vi "Transconductance state machine.vi"() -> ()   [LabVIEW 2016]
uses:
  <vilib>/Analysis/3filter.llb/Filter Passband Type.ctl
  <vilib>/Analysis/6fits.llb/Remove Outliers (Range).vi
  <vilib>/Analysis/3filter.llb/Chebyshev Filter (DBL).vi
  <vilib>/Analysis/NI_AALPro.lvlib
  <vilib>/Analysis/NI_AALBase.lvlib
  <vilib>/Analysis/NI_AAL_SigProc.lvlib
panel:
  in  "Tab Control 2":T1(tab)
  out "Conductance curve\nvertical line cut":cluster{dbl[], "Decimated Array":dbl[]}(graph)
  out "B field (T)":dbl
  out "Transcond curve\nhorizontal line cut":cluster{dbl[], dbl[]}(graph)
  out "Vsg (V)":dbl format="%#_6p"
  in  "Load data":bool
  in  "Refresh":bool
  in  "Tab Control":T2(tab)=enum."Flatten Transconductance"
  in  "index":T3={"N1 (x axis)"=3, "N2"=19, "N3"=4, "N4"=5, "V1"=8, "V2"=4, "V3"=10, "V4"=13, "CURRENT"=6, "Vsg"=1}
  in  "File or Folder Path":path=path "G:/My Drive/ansom/Data/MNK/SA03018F.20180426/3 - sweep B, Vsg lockin, superlattice"
  out "original cond":T4(graph)
  out "Comments":string="IGOR\nX// Date: 5/2/2018 10:25 PM\nX// B=0T to 18T, 0.03 T/min\nX// T=40mK\nX// sweep Vsg -10mV --> 60mV, 50uV step\nX// Vsg=1.1V\nX// \nX// lockin settings:\nX// time constant =100ms\nX// order=2\nX// Fs=13000\nX// #s=1000\nX// \nX// both\nX// \nX// lockin:\nX// 0: 4, voltage V+\nX// 1: 5,  current 50uV AC 270uV DC, 13 Hz\nX// 2: 7,voltage V-\nX// 3: 3, current, drain\nX// 4: 2,\nX// 5: 1, \nX// `INDEX`<WavesIndex_In_2>\n\nX//   <Side_Gate>1</Side_Gate>\n\nX//   <Current>6</Current>\n\nX//   <Voltage_1>8</Voltage_1>\n\nX//   <Voltage_2>4</Voltage_2>\n\nX//   <B_Field>3</B_Field>\n\nX//   <Voltage>true</Voltage>\n\nX// </WavesIndex_In_2>`INDEX`\n\n\n\n\n\n\n\n\n\n\n\n\n\n\n\n\n\n\n\n\n\n\n\n\n\n\n\n\n\n\n\n\n\n\n\n\n\n\n\n\n\n\n\n\n\n\n\n\n\n\n\n\n\n\n\n\n\n\nX \nX Display/R 'time.SA03018F.20180502.000001'\nX AppendToGraph 'Vsg.SA03018F.20180502.000001'\nX AppendToGraph 'T.SA03018F.20180502.000001'\nX AppendToGraph 'B.SA03018F.20180502.000001'\nX AppendToGraph 'X0.SA03018F.20180502.000001'\nX AppendToGraph 'Y0.SA03018F.20180502.000001'\nX AppendToGraph 'X1.SA03018F.20180502.000001'\nX AppendToGraph 'Y1.SA03018F.20180502.000001'\nX AppendToGraph 'X2.SA03018F.20180502.000001'\nX AppendToGraph 'Y2.SA03018F.20180502.000001'\nX AppendToGraph 'X3.SA03018F.20180502.000001'\nX AppendToGraph 'Y3.SA03018F.20180502.000001'\nX AppendToGraph 'X4.SA03018F.20180502.000001'\nX AppendToGraph 'Y4.SA03018F.20180502.000001'\nX AppendToGraph 'X5.SA03018F.20180502.000001'\nX AppendToGraph 'Y5.SA03018F.20180502.000001'\nX AppendToGraph 'B_rate.SA03018F.20180502.000001'\nX AppendToGraph 'R4t(e2/h).SA03018F.20180502.000001'\nX AppendToGraph 'axis1.SA03018F.20180502.000001'\nX AppendToGraph 'axis2.SA03018F.20180502.000001'\nX AppendToGraph '20.SA03018F.20180502.000001'\nX AppendToGraph '21.SA03018F.20180502.000001'\nX AppendToGraph '22.SA03018F.20180502.000001'\nX AppendToGraph '23.SA03018F.20180502.000001'\nX AppendToGraph '24.SA03018F.20180502.000001'\nX AppendToGraph '25.SA03018F.20180502.000001'\nX AppendToGraph '26.SA03018F.20180502.000001'\nX AppendToGraph '27.SA03018F.20180502.000001'\nX Label bottom \"x label\"\nX Label left \"y label\"\nX ModifyGraph rgb('time.SA03018F.20180502.000001')=(65280,0,0)\nX ModifyGraph rgb('Vsg.SA03018F.20180502.000001')=(65280,12288,0)\nX ModifyGraph rgb('T.SA03018F.20180502.000001')=(65280,24576,0)\nX ModifyGraph rgb('B.SA03018F.20180502.000001')=(65280,38400,0)\nX ModifyGraph rgb('X0.SA03018F.20180502.000001')=(65280,50688,0)\nX ModifyGraph rgb('Y0.SA03018F.20180502.000001')=(65280,62976,0)\nX ModifyGraph rgb('X1.SA03018F.20180502.000001')=(55808,65280,0)\nX ModifyGraph rgb('Y1.SA03018F.20180502.000001')=(43520,65280,0)\nX ModifyGraph rgb('X2.SA03018F.20180502.000001')=(29696,65280,0)\nX ModifyGraph rgb('Y2.SA03018F.20180502.000001')=(17408,65280,0)\nX ModifyGraph rgb('X3.SA03018F.20180502.000001')=(5120,65280,0)\nX ModifyGraph rgb('Y3.SA03018F.20180502.000001')=(0,65280,7168)\nX ModifyGraph rgb('X4.SA03018F.20180502.000001')=(0,65280,20992)\nX ModifyGraph rgb('Y4.SA03018F.20180502.000001')=(0,65280,33280)\nX ModifyGraph rgb('X5.SA03018F.20180502.000001')=(0,65280,45568)\nX ModifyGraph rgb('Y5.SA03018F.20180502.000001')=(0,65280,57856)\nX ModifyGraph rgb('B_rate.SA03018F.20180502.000001')=(0,60928,65280)\nX ModifyGraph rgb('R4t(e2/h).SA03018F.20180502.000001')=(0,47104,65280)\nX ModifyGraph rgb('axis1.SA03018F.20180502.000001')=(0,34816,65280)\nX ModifyGraph rgb('axis2.SA03018F.20180502.000001')=(0,22528,65280)\nX ModifyGraph rgb('20.SA03018F.20180502.000001')=(0,10240,65280)\nX ModifyGraph rgb('21.SA03018F.20180502.000001')=(2048,0,65280)\nX ModifyGraph rgb('22.SA03018F.20180502.000001')=(15872,0,65280)\nX ModifyGraph rgb('23.SA03018F.20180502.000001')=(28160,0,65280)\nX ModifyGraph rgb('24.SA03018F.20180502.000001')=(40448,0,65280)\nX ModifyGraph rgb('25.SA03018F.20180502.000001')=(52736,0,65280)\nX ModifyGraph rgb('26.SA03018F.20180502.000001')=(65280,0,64512)\nX ModifyGraph rgb('27.SA03018F.20180502.000001')=(65280,0,52224)\nX Legend/C/N=text0/J \"\\\\s('time.SA03018F.20180502.000001') time\\r\\\\s('Vsg.SA03018F.20180502.000001') Vsg\\r\\\\s('T.SA03018F.20180502.000001') T\\r\\\\s('B.SA03018F.20180502.000001') B\\r\\\\s('X0.SA03018F.20180502.000001') X0\\r\\\\s('Y0.SA03018F.20180502.000001') Y0\\r\\\\s('X1.SA03018F.20180502.000001') X1\\r\\\\s('Y1.SA03018F.20180502.000001') Y1\\r\\\\s('X2.SA03018F.20180502.000001') X2\\r\\\\s('Y2.SA03018F.20180502.000001') Y2\\r\\\\s('X3.SA03018F.20180502.000001') X3\\r\\\\s('Y3.SA03018F.20180502.000001') Y3\\r\\\\s('X4.SA03018F.20180502.000001') X4\\r\\\\s('Y4.SA03018F.20180502.000001') Y4\\r\\\\s('X5.SA03018F.20180502.000001') X5\\r\\\\s('Y5.SA03018F.20180502.000001') Y5\\r\\\\s('B_rate.SA03018F.20180502.000001') B_rate\\r\\\\s('R4t(e2/h).SA03018F.20180502.000001') R4t (e2/h)\\r\\\\s('axis1.SA03018F.20180502.000001') axis 1\\r\\\\s('axis2.SA03018F.20180502.000001') axis 2\"\nX ModifyGraph mirror(bottom)=1\nX ModifyGraph width=216\nX ModifyGraph height={Aspect,0.6}\nX ModifyGraph Log(bottom)=0\nX ModifyGraph Log(left)=0\nX \n"
  in  "offset":i32
  in  "length":i32=1000
  in  "conductance range":dbl[](array[numeric])=[-1.0, 20.0]
  in  "Filter?":bool=TRUE
  in  "low cutoff freq: fh 2":dbl=0.05 format="%0.2f"
  in  "restrict range?":bool=TRUE
  in  "dy/dx vs x":bool=TRUE
  in  "derivative points":dbl=20.0
  out "Cond intensity":dbl[][](graph)
  out "Conductance":T4(graph)
  in  "offset cond (horizontal)":dbl=0.001
  out "Transconductance":T4(graph)
  out "Transcond Intensity":dbl[][](graph)
  in  "offset trans (vertical)":dbl
  out "modified transconductance":T4(graph)
  in  "threshold":dbl=25.0 format="%0.2f"
  in  "width":i32=20 min=3
  in  "X Low":dbl=-0.1 format="%#_6p"
  in  "X High":dbl=0.1 format="%#_6p"
  out "Flattened Transconductance":dbl[][](graph)
  in  "manual offset array":dbl[](array[numeric])
  out "number of curves":i32
  in  "Stop":bool
  # "Conductance curve, select using cursor on transconductance \nintensity plot"
  # "choose N1 to be the B field, or other slow parameter\nfor intensity plots"
  # "creates conductnace plot\ny axis: current/(V1-V2)\nx axis: Vsg"
  # "To apply changes press the 'Refresh' button"
  # "Modify conductance data"
  # "Transconductnace derivative parameters"
  # "Peak finding parameters for \nflattening transconductance"
  # "Interpolating parameters"
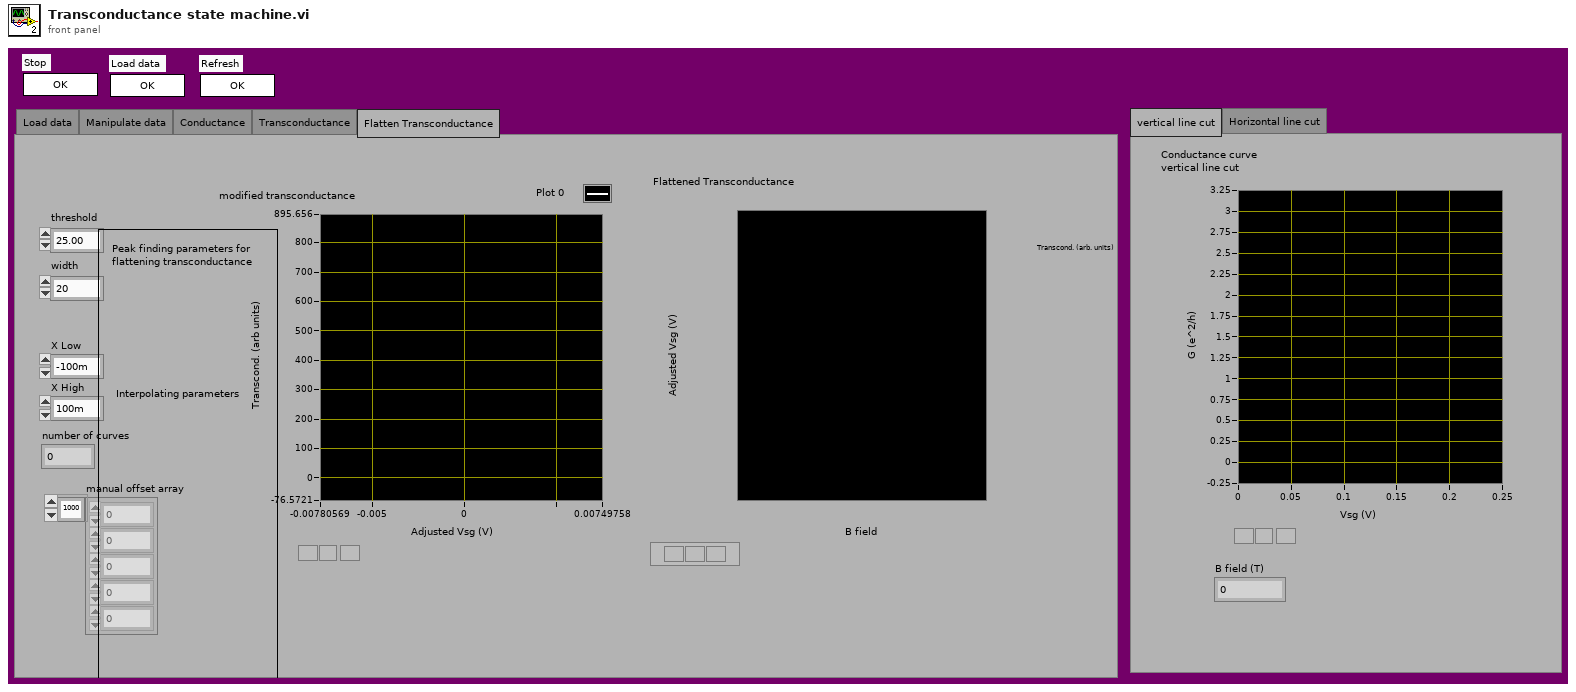
[diagram p1: front panel]
types:
  T1 = enum32{"vertical line cut", "Horizontal line cut"}
  T2 = enum32{"Load data", "Manipulate data", "Conductance", "Transconductance", "Flatten Transconductance"}
  T3 = cluster{"N1 (x axis)":i32, "N2":i32, "N3":i32, "N4":i32, "V1":i32, "V2":i32, "V3":i32, "V4":i32, "CURRENT":i32, "Vsg":i32}
  T4 = cluster{"Vfast":dbl[], "Decimated Array":dbl[]}[]
  T5 = enum32{"invalid app kind", "Development System", "Run Time System", "Student Edition", "Embedded LabVIEW", "Evaluation", "Custom"}
  T6 = enum32{"Invalid", "Standard", "Closed", "Hidden", "Minimized", "Maximized"}
  T7 = typedef "NI_AALBase.lvlib/Filter Passband Type.ctl" = enum32{"Lowpass", "Highpass", "Bandpass", "Bandstop"}
  T8 = cluster{"Core":cluster{"Current VI Reference":refnum<vi>, "Close Panel on Exit?":bool}, "Original Conductance":cluster{"Vfast":dbl[], "Decimated Array":dbl[]}[], "Modified Conductance":cluster{"Vfast":dbl[], "Decimated Array":dbl[]}[], "Transconductance":cluster{"Vfast":dbl[], "Decimated Array":dbl[]}[], "Modified Transconductance":cluster{"Vfast":dbl[], "Decimated Array":dbl[]}[], "Cond Intensity":dbl[][], "Transcond Intensity":dbl[][], "N Array":cluster{"N1":dbl, "N2":dbl, "N3":dbl, "N4":dbl}[], "N1 (B field)":dbl[], "Vsg offset and mult":cluster{dbl, dbl}, "B offset and mult":cluster{dbl, dbl}, "number of curves":i32, "cursor plot":i32, "curson index":i32}
  T9 = cluster{"N1":dbl, "N2":dbl, "N3":dbl, "N4":dbl}[]
  T10 = cluster{"Current VI Reference":refnum<vi>, "Close Panel on Exit?":bool}
  T11 = typedef "LVOffsetAndMultiplierTypeDef.ctl" = cluster{"Offset":dbl, "Multiplier":dbl}
  T12 = cluster{"Decimated Array":dbl[], "Decimated Array":dbl[]}
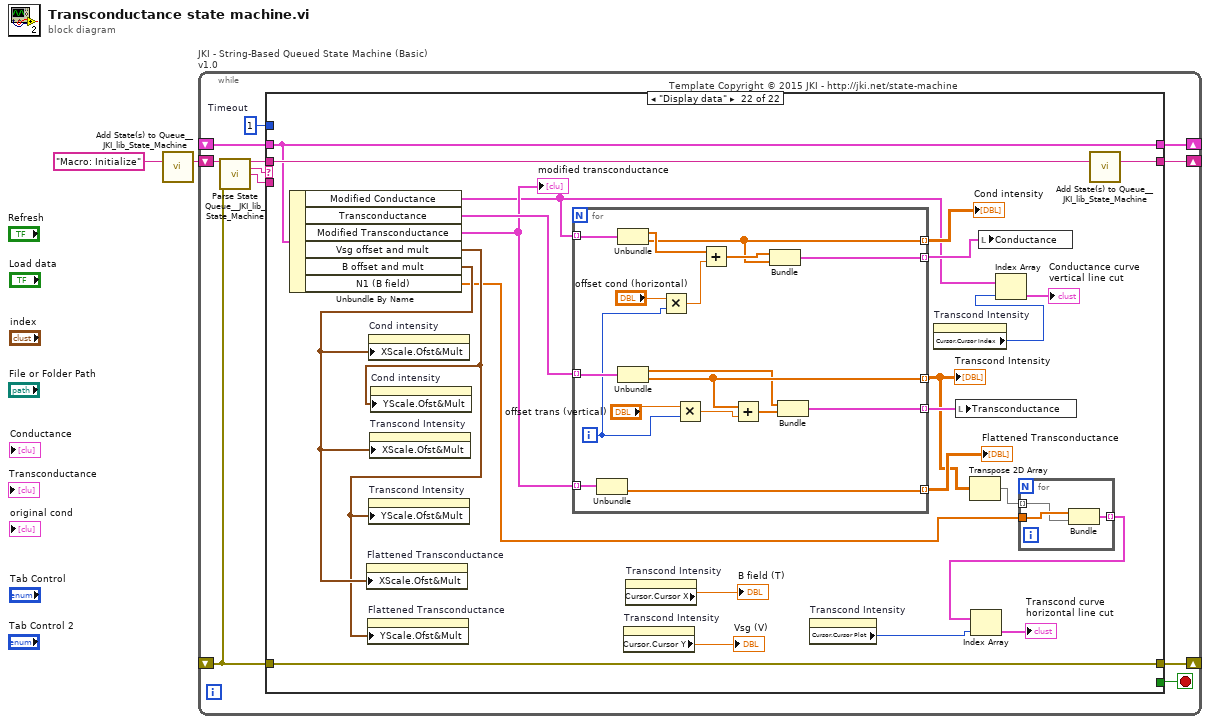
[diagram p0: block diagram]
diagram:
  n1 = call <vilib>:"Add State(s) to Queue__JKI_lib_State_Machine.vi"("State(s) in (\"\")"="Macro: Initialize") -> ("States Out"=w2:string)  [unwired: 14 in]
  n2 = while "JKI - String-Based Queued State Machine (Basic) v1.0" {
    shift-right: [w6] -> _
    shift-left: _ -> [w5]
    shift-right: [w9] -> _
    shift-left: _ -> [w3]
    shift-right: [w8] -> _
    shift-left: w2 -> [w10]
    stop <- w7 stop-if-true
    w4 = 1  # Timeout
    # "Template Copyright © 2015 JKI - http://jki.net/state-machine"
    n3 = call <vilib>:"Parse State Queue__JKI_lib_State_Machine.vi"("State Queue"=w10, "Error In (no error)"=w3) -> ("Remaining States"=w12:string, "Current State"=w13:string, "Arguments"=w11:string)  [unwired: 11 in]
    n4 = case shown="\"Display data\"" w13 {
      selector: w13 -> [_ _ w82 _ _ _ _ _ _ _ _ _ _ _ _ _ _ _ _ _ _ _]
      tunnel: w12 -> [w20 w81 w86 w104 w110 w115 w119 w137 w143 w147 w155 w161 w172 w198 w203 w213 w217 w256 w269 w298 w316 w357]
      tunnel: w11 -> [_ _ _ _ _ _ _ _ _ _ _ w156 w166 _ _ _ _ _ _ _ _ _]
      tunnel: w5 -> [w18 w78 w84 w95 w107 w113 w116 _ w138 w144 w152 w159 w168 w195 w200 w210 w214 w223 w261 w294 w313 w354]
      tunnel: [w17 w79 w88 w101 errorcluster {"status"=FALSE, "code"=0, "source"=""} ("error out") w112 w117 w134 w139 w145 w153 w157 w169 w196 w201 w211 w215 w254 w267 w296 w314 w355] -> w9
      tunnel: w3 -> [w16 w79 w87 w101 w106 w112 w117 w134 w140 w145 w153 w158 w170 w196 w201 w211 w215 w254 w267 w296 w314 w355]
      tunnel: [w19 w80 w85 w103 w109 w114 w118 w136 w142 w146 w154 w160 w171 w197 w202 w212 w216 w255 w268 w297 w315 w356] -> w8
      tunnel: [_ _ _ _ _ TRUE _ _ _ _ _ _ _ _ _ _ _ _ _ _ _ _] -> w7
      tunnel: [w15 w78 w84 w102 w107 w113 w116 w135 w138 w144 w150 w159 w168 w195 w200 w210 w214 w251 w259 w292 w312 w354] -> w6
      tunnel: w4 -> [w14 _ _ _ _ _ _ _ _ _ _ _ _ _ _ _ _ _ _ _ _ _]
      frame "", "Event Structure", "Idle" {
        # "executes when the state queue is empty"
        n5 = event shown="[3] \"Refresh\": Value Change" {
          selector: _ -> [_ _ _ _ _ _ _ _]
          dyn-events: _ -> [_ _ _ _ _ _ _ _]
          timeout: w14 -> [_ _ _ _ _ _ _ _]
          tunnel: w20 -> [w30 w35 w40 w45 w46 w56 w69 w77]
          tunnel: [w29 w34 w39 w44 w47 w55 w68 w76] -> w19
          tunnel: w18 -> [w26 w32 w37 w42 w49 w57 w67 w74]
          tunnel: [w28 w33 w38 w43 w48 w54 w62 w75] -> w17
          tunnel: w16 -> [w28 w33 w38 w43 w48 w54 w62 w75]
          tunnel: [w25 w32 w37 w42 w49 w57 w67 w74] -> w15
          event Timeout {
            n6 = event-data() -> ()  [unwired: 1 in, 1 out]
            n7 = local read "original cond"() -> (w22:T4)
            n8 = property on="Transcond Intensity" class="IntGraph (strict)"() -> ("Cursor.Cursor Index"=w23:i32)  [unwired: 2 in, 2 out]
            n9 = property on="Transcond Intensity" class="IntGraph (strict)"() -> ("Cursor.Cursor Plot"=w24:i32)  [unwired: 2 in, 2 out]
            n10 = Array Size(array=w22) -> (size(s)=w21:i32)
            n11 = Bundle By Name(cluster=w26, "cursor plot"=w24, "curson index"=w23, "number of curves"=w21) -> (w25:T8)
            n12 = call <vilib>:"Add State(s) to Queue__JKI_lib_State_Machine.vi"("State(s) in (\"\")"=w30, "State(s) at Back (\"\")"="Display data" ("State(s) at Back (\"\")")) -> ("States Out"=w29:string)  [unwired: 13 in]
          }
          event "Stop": Value Change {
            # "Exit Button Value Change (pressed) Event\n(this executes Macro: Exit to terminate the VI)"
            n13 = event-data() -> ()  [unwired: 1 in, 1 out]
            n14 = call <vilib>:"Add State(s) to Queue__JKI_lib_State_Machine.vi"("State(s) in Front (\"\")"="Macro: Exit", "State(s) in (\"\")"=w35) -> ("States Out"=w34:string)  [unwired: 13 in]
          }
          event "Load data": Value Change {
            # "Load data using 'Calculate conductance ITX.vi'\n\nmust set the folder path and the index"
            n15 = event-data() -> ()  [unwired: 1 in, 1 out]
            n16 = call <vilib>:"Add State(s) to Queue__JKI_lib_State_Machine.vi"("State(s) in Front (\"\")"="Load data", "State(s) in (\"\")"=w40) -> ("States Out"=w39:string)  [unwired: 13 in]
          }
          event "Refresh": Value Change {
            # "Refresh graphs with any changes in manipulate data tab\n\nwill also display the data in the 'original cond' graph if no\nnew data has been loaded since starting the program"
            n17 = event-data() -> ()  [unwired: 1 in, 1 out]
            n18 = call <vilib>:"Add State(s) to Queue__JKI_lib_State_Machine.vi"("State(s) in Front (\"\")"="Manipulate data", "State(s) in (\"\")"=w45) -> ("States Out"=w44:string)  [unwired: 13 in]
          }
          event "Flattened Transconductance": Cursor Move {
            n19 = event-data() -> ()  [unwired: 1 in, 9 out]
            n20 = property on="Flattened Transconductance" class="IntGraph (strict)"() -> ("Cursor.Cursor Index"=w51:i32, "Cursor.Cursor Plot"=w50:i32)  [unwired: 2 in, 2 out]
            n21 = property on="Transcond Intensity" class="IntGraph (strict)"("Cursor.Cursor Index"=w51, "Cursor.Cursor Plot"=w50) -> ()  [unwired: 2 in, 2 out]
            n22 = call <vilib>:"Add State(s) to Queue__JKI_lib_State_Machine.vi"("State(s) in (\"\")"=w46) -> ("States Out"=w47:string)  [unwired: 14 in]
          }
          event "Cond intensity": Cursor Move {
            n23 = event-data() -> ()  [unwired: 1 in, 9 out]
            n24 = property on="Cond intensity" class="IntGraph (strict)"() -> ("Cursor.Cursor Index"=w53:i32, "Cursor.Cursor Plot"=w52:i32)  [unwired: 2 in, 2 out]
            n25 = property on="Transcond Intensity" class="IntGraph (strict)"("Cursor.Cursor Index"=w53, "Cursor.Cursor Plot"=w52) -> ()  [unwired: 2 in, 2 out]
            n26 = call <vilib>:"Add State(s) to Queue__JKI_lib_State_Machine.vi"("State(s) in (\"\")"=w56) -> ("States Out"=w55:string)  [unwired: 14 in]
          }
          event "Transcond Intensity": Cursor Move {
            # "Change visible tab in line cut tab control when the cursor on the transconductance intensity plot is moved\nmoving the vertical cursor shows the vertical line cut, moving the horizontal cursor shows the horizontal line cut"
            n27 = event-data() -> ("CursIdx"=w63:i32, "PlotIdx"=w64:i32)  [unwired: 1 in, 7 out]
            n28 = Unbundle By Name(w67) -> ("curson index"=w66:i32, "cursor plot"=w65:i32)
            n29 = Not Equal?(x=w66, y=w63) -> (x != y?=w61:bool)
            n30 = Not Equal?(x=w65, y=w64) -> (x != y?=w60:bool)
            n31 = And(x=w61, y=w60) -> (x .and. y?=w59:bool)
            n32 = case shown="True" w59 {
              tunnel: [T1."vertical line cut" ("Tab Control 2") T1."Horizontal line cut" ("Tab Control 2")] -> w58
              frame False {
              }
              frame True {
              }
            }
            n33 = local write "Tab Control 2"(w58) -> ()
            n34 = call <vilib>:"Add State(s) to Queue__JKI_lib_State_Machine.vi"("State(s) in (\"\")"=w69) -> ("States Out"=w68:string)  [unwired: 14 in]
          }
          event Panel Close? {
            # "Discard the event because we'll close the front panel ourselves in Macro: Exit"
            # "Close Panel button (pressed) Event\n(this executes Macro: Exit to terminate the VI)"
            n35 = event-data() -> ()  [unwired: 1 in, 1 out]
            n36 = call <vilib>:"Add State(s) to Queue__JKI_lib_State_Machine.vi"("State(s) in Front (\"\")"="Macro: Exit", "State(s) in (\"\")"=w77) -> ("States Out"=w76:string)  [unwired: 13 in]
            n37 = event-data("Discard?"=TRUE) -> ()  [unwired: 1 in, 1 out]
          }
        }
      }
      frame "---------- Core ----------" {
        # "Do not put any code in this frame.\n(it is a separator no-op)"
        n38 = call <vilib>:"Add State(s) to Queue__JKI_lib_State_Machine.vi"("State(s) in (\"\")"=w81) -> ("States Out"=w80:string)  [unwired: 14 in]
      }
      frame Default {
        w91 = 42 items=["No error", "Argument error", "Memory is full", "Out of zone", "End of file", "File already open", "Generic file I/O error", "File not found", "File permission error", "Disk is full", "Duplicate path", "Too many files open", "System feature not enabled", "Resource file not found", "Cannot add resource", "Resource not found", "Image not found", "Image memory error", "Pen does not exist", "Config type invalid", "Config token not found", "Config parse error", "Config memory error", "Bad external code format", "Bad external code offset", "External code not present", "Null window", "Destroy window error", "Null menu", "Print aborted", "Bad print record", "Print driver error", "Windows error during printing", "Memory error during printing", "Print dialog error", "Generic print error", "Invalid device refnum", "Device not found", "Device parameter error", "Device unit error", "Cannot open device", "Device call aborted", "Generic error", "Cancelled by user", "Object ID too low", "Object ID too high", "Object not in heap", "Unknown heap", "Unknown object (invalid DefProc)", "Unknown object (DefProc not in table)", "Message out of range", "Invalid (null) method", "Unknown message", "Manager call not supported", "Bad address", "Network operation in progress", "Network operation timed out", "Connection is busy", "Network attribute not supported", "Network error", "Address in use", "System out of memory", "Connection aborted", "Connection refused", "Not connected", "Already connected", "Connection closed", "Initialization error (interapplication manager)", "Bad occurrence", "Wait on unbound occurrence handler", "Occurrence queue overflow", "Datalog type conflict", "Unused", "Unrecognized type (interapplication manager)", "Memory corrupt", "Failed to make temporary DLL", "Old CIN version", "Drag socket not found", "Failed to load drop-object", "Failed to register OLE object", "Failed to release OLE object", "Format specifier type mismatch", "Unknown format specifier", "Too few format specifiers", "Too many format specifiers", "Scan failed", "Newer CIN version", "Error converting to variant", "Runtime menu error", "Password tampered", "Variant attribute not found", "Incompatible variant data type", "Event data is not available", "Event Store is not present", "Occurrence is not found", "Event Queue is not created", "Event info is not available", "Refnum passed is NULL", "Error retrieving Class GUID", "Error retrieving CoClass GUID", "Error retrieving TypeLib GUID.", "Bad built application magic bytes.", "Specific driver is different from the specific driver associated with the Logical Name.", "There is no session opened to the class driver.", "Max Error", "MAX - Error with config objects", "MAX - Error loading configuration", "MAX - Group not supported"]
        # "Current State"
        # "Do not delete, rename, or modify this frame.\n(this is used to capture unhandled states and typos)"
        # "Handle mistyped state name (developer tool)"
        n39 = Format Into String(format string="Software Exception: Unhandled State \"%s\"." ("message"), error in=w87, w82) -> (resulting string=w90:string, error out=w89:errorcluster)  [unwired: 1 in]
        n40 = call <vilib>:"Error Cluster From Error Code.vi"("show call chain? (False)"=TRUE, "error in (no error)"=w89, "error message (\"\")"=w90, "error code (0)"=w91) -> ("error out"=w88:errorcluster)  [unwired: 5 in]
        n41 = call <vilib>:"Add State(s) to Queue__JKI_lib_State_Machine.vi"("State(s) in (\"\")"=w86) -> ("States Out"=w85:string)  [unwired: 14 in]
      }
      frame "Initialize Core Data" {
        # "Do not delete, rename, or modify this frame.\n(this is used to determine panel behavior on exit)"
        # "originally closed?"
        # "exe?"
        # "If panel starts closed or is an EXE, then close it when we exit"
        n42 = property class="VI"() -> ("Front Panel.Open"=w100:bool)  [unwired: 2 in, 2 out]
        n43 = property class="App"() -> ("App.Kind"=w99:T5)  [unwired: 2 in, 2 out]
        n44 = control-ref of="Current VI Reference"() -> (w93:refnum<vi>)
        n45 = Not(x=w100) -> (.not. x?=w97:bool)
        n46 = Equal?(x=w99, y=T5."Run Time System" ("Application:Kind")) -> (x = y?=w96:bool)
        n47 = Or(x=w97, y=w96) -> (x .or. y?=w94:bool)
        n48 = Bundle By Name(cluster=w95, "Core.Current VI Reference"=w93, "Core.Close Panel on Exit?"=w94) -> (w102:T8)
        n49 = call <vilib>:"Add State(s) to Queue__JKI_lib_State_Machine.vi"("State(s) in (\"\")"=w104) -> ("States Out"=w103:string)  [unwired: 14 in]
      }
      frame "Error Handler" {
        # "Unhandled Error -- Display it"
        # "Handle any errors here.\nYou can also output any states to clean-up after errors occur"
        # "Clear error"
        n50 = call <vilib>:"General Error Handler.vi"("error in (no error)"=w106) -> ()  [unwired: 10 in, 5 out]
        n51 = call <vilib>:"Add State(s) to Queue__JKI_lib_State_Machine.vi"("State(s) in Front (\"\")"="/* Post Error States", "State(s) in (\"\")"=w110) -> ("States Out"=w109:string)  [unwired: 13 in]
      }
      frame "Exit" {
        # "Do not put any code in this frame.\n(No errors that occur here will be handled.)"
        n52 = call <vilib>:"Add State(s) to Queue__JKI_lib_State_Machine.vi"("State(s) in (\"\")"=w115) -> ("States Out"=w114:string)  [unwired: 14 in]
      }
      frame "---------- Data ----------" {
        # "Do not put any code in this frame.\n(It is a separator no-op. You can make a copy of this frame to create a new Data frame)"
        n53 = call <vilib>:"Add State(s) to Queue__JKI_lib_State_Machine.vi"("State(s) in (\"\")"=w119) -> ("States Out"=w118:string)  [unwired: 14 in]
      }
      frame "Data: Initialize" {
        w120 = 0  # curson index
        w121 = 0  # cursor plot
        w122 = T4 []  # Modified Transconductance
        w123 = 0  # number of curves
        w124 = cluster{dbl, dbl} {0.0, 0.0}  # B offset and mult
        w125 = cluster{dbl, dbl} {0.0, 0.0}  # Vsg offset and mult
        w126 = dbl[] []  # N1 (B field)
        w127 = T4 []  # Modified Conductance
        w128 = T9 [{"N1"=0.1054, "N2"=0.0, "N3"=7.167371706088133e-06, "N4"=1.53337376832391e-06}, {"N1"=0.2744, "N2"=0.0, "N3"=7.516017465840743e-06, "N4"=1.870780961155766e-06}, {"N1"=0.4429, "N2"=0.0, "N3"=7.164956665698316e-06, "N4"=2.24365763977575e-06}, {"N1"=0.6118, "N2"=0.0, "N3"=7.47503008732585e-06, "N4"=2.509786953376164e-06}, {"N1"=0.78, "N2"=0.0, "N3"=7.582119269367365e-06, "N4"=1.865776048611999e-06}, {"N1"=0.9496, "N2"=0.0, "N3"=7.367991857506643e-06, "N4"=2.698521756661702e-06}, {"N1"=1.1176, "N2"=0.0, "N3"=7.227789507339006e-06, "N4"=2.57461130832219e-06}, {"N1"=1.2843, "N2"=0.0, "N3"=7.066841533109455e-06, "N4"=3.048492296414582e-06}, {"N1"=1.4544, "N2"=0.0, "N3"=6.956050970108828e-06, "N4"=3.922270862071821e-06}, {"N1"=1.6231, "N2"=0.0, "N3"=7.236120895401367e-06, "N4"=3.382292471609201e-06}, {"N1"=1.7923, "N2"=0.0, "N3"=7.409928531135188e-06, "N4"=2.980502224034656e-06}, {"N1"=1.9608, "N2"=0.0, "N3"=7.465240274926555e-06, "N4"=2.567980193012299e-06}, {"N1"=2.1296, "N2"=0.0, "N3"=7.67996705698243e-06, "N4"=2.820594776222847e-06}, {"N1"=2.2974, "N2"=0.0, "N3"=7.462806473700619e-06, "N4"=3.043330294253364e-06}, {"N1"=2.4668, "N2"=0.0, "N3"=7.436808347763807e-06, "N4"=2.755707470732885e-06}, {"N1"=2.6348, "N2"=0.0, "N3"=6.62119487806683e-06, "N4"=3.938204565752024e-06}, {"N1"=2.8044, "N2"=0.0, "N3"=7.474110207381518e-06, "N4"=2.685132266272008e-06}, {"N1"=2.9727, "N2"=0.0, "N3"=7.467721317681889e-06, "N4"=2.490711666292731e-06}, {"N1"=3.1413, "N2"=0.0, "N3"=7.373756967263423e-06, "N4"=3.233877080828954e-06}, {"N1"=3.3108, "N2"=0.0, "N3"=7.665479000670658e-06, "N4"=2.656474229977507e-06}, {"N1"=3.4787, "N2"=0.0, "N3"=7.590986063837561e-06, "N4"=2.372468698283599e-06}, {"N1"=3.6474, "N2"=0.0, "N3"=7.403426727936138e-06, "N4"=2.492719733694041e-06}, {"N1"=3.8169, "N2"=0.0, "N3"=7.673375229594714e-06, "N4"=2.203309425429715e-06}, {"N1"=3.9853, "N2"=0.0, "N3"=7.235339121315365e-06, "N4"=2.455197981754483e-06}, {"N1"=4.1517, "N2"=0.0, "N3"=7.588783683002382e-06, "N4"=2.171945449692774e-06}, {"N1"=4.3221, "N2"=0.0, "N3"=7.448410925151985e-06, "N4"=2.89278994654584e-06}, {"N1"=4.4909, "N2"=0.0, "N3"=7.559811002403063e-06, "N4"=2.32906566750442e-06}, {"N1"=4.6597, "N2"=0.0, "N3"=7.589944875648538e-06, "N4"=2.522315779577562e-06}, {"N1"=4.828, "N2"=0.0, "N3"=7.486560787096485e-06, "N4"=2.673968837700548e-06}, {"N1"=4.9975, "N2"=0.0, "N3"=7.764068992589737e-06, "N4"=2.470810112270278e-06}, {"N1"=5.1656, "N2"=0.0, "N3"=7.515430091426793e-06, "N4"=2.347750168384078e-06}, {"N1"=5.3343, "N2"=0.0, "N3"=7.61778177581086e-06, "N4"=2.441280739349988e-06}, {"N1"=5.5028, "N2"=0.0, "N3"=7.648092365254961e-06, "N4"=2.50884391552613e-06}, {"N1"=5.6718, "N2"=0.0, "N3"=7.607187802074639e-06, "N4"=2.479224506195392e-06}, {"N1"=5.8408, "N2"=0.0, "N3"=7.675790190344634e-06, "N4"=2.243726367409315e-06}, {"N1"=6.0093, "N2"=0.0, "N3"=7.5989905280867e-06, "N4"=2.339493694595715e-06}, {"N1"=6.1776, "N2"=0.0, "N3"=7.946377320613181e-06, "N4"=2.179171604450671e-06}, {"N1"=6.3464, "N2"=0.0, "N3"=7.788145582711778e-06, "N4"=1.980962373666305e-06}, {"N1"=6.5143, "N2"=0.0, "N3"=7.613597487476077e-06, "N4"=2.305590643717492e-06}, {"N1"=6.6841, "N2"=0.0, "N3"=7.704173394418159e-06, "N4"=2.229928539054291e-06}, {"N1"=6.8524, "N2"=0.0, "N3"=7.719187746028896e-06, "N4"=1.959910122360407e-06}, {"N1"=7.0199, "N2"=0.0, "N3"=7.54069778807839e-06, "N4"=2.119395007811887e-06}, {"N1"=7.1892, "N2"=0.0, "N3"=7.780578976603794e-06, "N4"=2.065252716472169e-06}, {"N1"=7.359, "N2"=0.0, "N3"=7.850755995736213e-06, "N4"=2.026777225217505e-06}, {"N1"=7.5271, "N2"=0.0, "N3"=7.948557406193015e-06, "N4"=2.288103766199132e-06}, {"N1"=7.6959, "N2"=0.0, "N3"=7.516853899196371e-06, "N4"=1.934437391177251e-06}, {"N1"=7.8642, "N2"=0.0, "N3"=7.636061465147594e-06, "N4"=2.309715289559359e-06}, {"N1"=8.0328, "N2"=0.0, "N3"=7.633733901431548e-06, "N4"=2.130290776686087e-06}, {"N1"=8.2016, "N2"=0.0, "N3"=7.731748664793311e-06, "N4"=2.089276305545186e-06}, {"N1"=8.3703, "N2"=0.0, "N3"=7.724840467667309e-06, "N4"=2.368731238393298e-06}, {"N1"=8.5396, "N2"=0.0, "N3"=7.765278384713542e-06, "N4"=1.945694195098239e-06}, {"N1"=8.7073, "N2"=0.0, "N3"=7.74873723912328e-06, "N4"=2.207113540673977e-06}, {"N1"=8.8765, "N2"=0.0, "N3"=7.855372955985145e-06, "N4"=1.962585706208197e-06}, {"N1"=9.0455, "N2"=0.0, "N3"=7.843310241373774e-06, "N4"=1.925552700333144e-06}, {"N1"=9.2141, "N2"=0.0, "N3"=7.86110382470724e-06, "N4"=2.081739111499381e-06}, {"N1"=9.3828, "N2"=0.0, "N3"=7.872060865040445e-06, "N4"=2.103890420690471e-06}, {"N1"=9.5511, "N2"=0.0, "N3"=7.577362880483975e-06, "N4"=3.032802004782522e-06}, {"N1"=9.7204, "N2"=0.0, "N3"=7.687842862590589e-06, "N4"=1.874148578396659e-06}, {"N1"=9.8887, "N2"=0.0, "N3"=8.061821348792517e-06, "N4"=1.394385993232741e-06}, {"N1"=10.0569, "N2"=0.0, "N3"=7.583223692545615e-06, "N4"=1.697687019205293e-06}, {"N1"=10.2263, "N2"=0.0, "N3"=7.959425651648591e-06, "N4"=1.719530895423454e-06}, {"N1"=10.3947, "N2"=0.0, "N3"=8.104826950424347e-06, "N4"=2.217009600034041e-06}, {"N1"=10.5631, "N2"=0.0, "N3"=8.092309435913141e-06, "N4"=1.86506523651042e-06}, {"N1"=10.7318, "N2"=0.0, "N3"=7.8911784041579e-06, "N4"=1.760112429967946e-06}, {"N1"=10.9009, "N2"=0.0, "N3"=7.96909852408623e-06, "N4"=1.66698686793123e-06}, {"N1"=11.0691, "N2"=0.0, "N3"=8.065608528600414e-06, "N4"=1.725471834153319e-06}, {"N1"=11.2379, "N2"=0.0, "N3"=8.155864753688254e-06, "N4"=4.665050563001727e-07}, {"N1"=11.407, "N2"=0.0, "N3"=7.80706842968668e-06, "N4"=1.460679749566241e-06}, {"N1"=11.5756, "N2"=0.0, "N3"=8.12897937207956e-06, "N4"=1.587939803265357e-06}, {"N1"=11.741, "N2"=0.0, "N3"=8.27251103469089e-06, "N4"=1.252388215033951e-06}, {"N1"=11.9126, "N2"=0.0, "N3"=7.797849423968604e-06, "N4"=1.267926363181601e-06}, {"N1"=12.0812, "N2"=0.0, "N3"=8.365431522458954e-06, "N4"=2.092208615272172e-09}, {"N1"=12.2499, "N2"=0.0, "N3"=8.039080769849434e-06, "N4"=9.836766439170422e-07}, {"N1"=12.4185, "N2"=0.0, "N3"=7.907582712890951e-06, "N4"=8.989608522161535e-07}, {"N1"=12.5874, "N2"=0.0, "N3"=8.274090537851438e-06, "N4"=9.664113986898211e-07}, {"N1"=12.756, "N2"=0.0, "N3"=7.839858031313029e-06, "N4"=6.065212034273762e-07}, {"N1"=12.9244, "N2"=0.0, "N3"=8.463881119681138e-06, "N4"=-4.136656659107811e-07}, {"N1"=13.0939, "N2"=0.0, "N3"=8.248317658130382e-06, "N4"=3.8802144716701056e-07}, {"N1"=13.2622, "N2"=0.0, "N3"=8.18069446636197e-06, "N4"=4.001100073970894e-07}, {"N1"=13.4308, "N2"=0.0, "N3"=7.946584223789573e-06, "N4"=4.854531765921596e-07}, {"N1"=13.5989, "N2"=0.0, "N3"=8.256171773806876e-06, "N4"=7.718940191013025e-08}, {"N1"=13.7683, "N2"=0.0, "N3"=8.357762676340478e-06, "N4"=-4.766689453610121e-07}, {"N1"=13.9361, "N2"=0.0, "N3"=8.112662582615276e-06, "N4"=4.696250710037667e-08}, {"N1"=14.1046, "N2"=0.0, "N3"=8.277448925942084e-06, "N4"=1.5985023049004504e-07}, {"N1"=14.2741, "N2"=0.0, "N3"=8.336889123617748e-06, "N4"=-2.0452091750021353e-07}, {"N1"=14.4421, "N2"=0.0, "N3"=8.30998027275276e-06, "N4"=4.5720936631723534e-08}, {"N1"=14.6088, "N2"=0.0, "N3"=8.29428838756584e-06, "N4"=-6.505469695250185e-07}, {"N1"=14.7799, "N2"=0.0, "N3"=8.385821104349947e-06, "N4"=-1.3494022655079468e-07}, {"N1"=14.9477, "N2"=0.0, "N3"=8.153057627152194e-06, "N4"=-3.459524396899026e-07}, {"N1"=15.1168, "N2"=0.0, "N3"=8.227366250614983e-06, "N4"=-1.2248894911569274e-07}, {"N1"=15.2855, "N2"=0.0, "N3"=8.445291874318747e-06, "N4"=-3.92114080863001e-07}, {"N1"=15.4543, "N2"=0.0, "N3"=8.32471765192864e-06, "N4"=-5.0620283647846016e-08}, {"N1"=15.6228, "N2"=0.0, "N3"=8.527397645132e-06, "N4"=-8.537202873107685e-07}, {"N1"=15.7909, "N2"=0.0, "N3"=8.397769046079376e-06, "N4"=-8.032897159765025e-07}, {"N1"=15.9596, "N2"=0.0, "N3"=8.548282390442658e-06, "N4"=-7.548173180977796e-07}, {"N1"=16.1276, "N2"=0.0, "N3"=8.419128550887185e-06, "N4"=-7.633414405502411e-07}, {"N1"=16.2972, "N2"=0.0, "N3"=8.415501486100044e-06, "N4"=-1.285585105550623e-06}, {"N1"=16.4645, "N2"=0.0, "N3"=8.600954461689525e-06, "N4"=-1.312315767726753e-06}, {"N1"=16.6337, "N2"=0.0, "N3"=8.593219192247852e-06, "N4"=-9.612729610059892e-07}, {"N1"=16.8019, "N2"=0.0, "N3"=8.389546202306117e-06, "N4"=-9.411302314844897e-07}, {"N1"=16.9709, "N2"=0.0, "N3"=8.71566870861619e-06, "N4"=-1.17801856081449e-06}, {"N1"=17.1383, "N2"=0.0, "N3"=8.425705561859544e-06, "N4"=-1.128343590270702e-06}, {"N1"=17.3074, "N2"=0.0, "N3"=8.712433922967295e-06, "N4"=-1.49946252612336e-06}, {"N1"=17.4742, "N2"=0.0, "N3"=8.790090932572884e-06, "N4"=-1.346827964006174e-06}, {"N1"=17.6436, "N2"=0.0, "N3"=8.704668257768896e-06, "N4"=-1.270644334526553e-06}, {"N1"=17.812, "N2"=0.0, "N3"=8.643630301112523e-06, "N4"=-1.240804614481721e-06}, {"N1"=17.9808, "N2"=0.0, "N3"=8.593810256963035e-06, "N4"=-1.493504631387627e-06}, {"N1"=18.0004, "N2"=0.0, "N3"=8.77741280386506e-06, "N4"=-1.330698644381706e-06}]  # N Array
        w129 = dbl[][] []  # Transcond Intensity
        w130 = dbl[][] []  # Cond Intensity
        w131 = T4 []  # Transconductance
        w132 = T4 []  # Original Conductance
        w133 = T10 {"Current VI Reference"=refnum, "Close Panel on Exit?"=FALSE}  # Core
        # "Initialize the shift-register data, here.\n(data names are defined by what you wire into the bundle function)"
        n54 = call <vilib>:"Add State(s) to Queue__JKI_lib_State_Machine.vi"("State(s) in (\"\")"=w137) -> ("States Out"=w136:string)  [unwired: 14 in]
        n55 = Bundle("Core"=w133, "Original Conductance"=w132, "Modified Conductance"=w127, "Transconductance"=w131, "Modified Transconductance"=w122, "Cond Intensity"=w130, "Transcond Intensity"=w129, "N Array"=w128, "N1 (B field)"=w126, "Vsg offset and mult"=w125, "B offset and mult"=w124, "number of curves"=w123, "cursor plot"=w121, "curson index"=w120) -> (w135:T8)  [unwired: 1 in]
      }
      frame "Data: Cleanup" {
        # "Cleanup any data and references, here.\n(this is called automatically, by the Macro: Exit)"
        n56 = Unbundle By Name(w138) -> ("Core.Current VI Reference"=w141:refnum<vi>)
        n57 = Close Reference(reference=w141, error in (no error)=w140) -> (error out=w139:errorcluster)
        n58 = call <vilib>:"Add State(s) to Queue__JKI_lib_State_Machine.vi"("State(s) in (\"\")"=w143) -> ("States Out"=w142:string)  [unwired: 14 in]
      }
      frame "---------- UI ----------" {
        # "Do not put any code in this frame.\n(It is a separator no-op. You can make a copy of this frame to create a new UI frame)"
        n59 = call <vilib>:"Add State(s) to Queue__JKI_lib_State_Machine.vi"("State(s) in (\"\")"=w147) -> ("States Out"=w146:string)  [unwired: 14 in]
      }
      frame "UI: Initialize" {
        n60 = property on="Transcond Intensity" class="IntGraph (strict)"() -> ("XScale.Ofst&Mult"=w149:T11)  [unwired: 2 in, 2 out]
        n61 = property on="Transcond Intensity" class="IntGraph (strict)"() -> ("YScale.Ofst&Mult"=w148:T11)  [unwired: 2 in, 2 out]
        n62 = local read "original cond"() -> (w151:T4)
        n63 = Bundle By Name(cluster=w152, "Original Conductance"=w151, "Vsg offset and mult"=w148, "B offset and mult"=w149) -> (w150:T8)
        n64 = call <vilib>:"Add State(s) to Queue__JKI_lib_State_Machine.vi"("State(s) in (\"\")"=w155) -> ("States Out"=w154:string)  [unwired: 14 in]
      }
      frame "UI: Cursor Set" {
        # "Argument"
        # "Set and Unset Cursor Busy.\n(Usage: \"UI: Cursor Set >> Busy|Idle\")"
        n65 = case shown="\"Idle\", Default" w156 {
          tunnel: w158 -> [w163 w165]
          tunnel: [w162 w164] -> w157
          frame "Idle", Default {
            n66 = call <vilib>:"Unset Busy.vi"("error in (no error)"=w163) -> ("error out"=w162:errorcluster)  [unwired: 10 in]
          }
          frame "Busy" {
            n67 = call <vilib>:"Set Busy.vi"("error in (no error)"=w165) -> ("error out"=w164:errorcluster)  [unwired: 9 in, 1 out]